vi "CRYO_MASTER_FULL_dev.vi"() -> ()   [LabVIEW 2017] (continued)
          }
          frame #2 {
            n644 = Search 1D Array(1D array=w1301, element="3He inlet pressure") -> (index of element=w1299:i32)  [unwired: 1 in]
            n645 = Index Array(array=w1300, index=w1299) -> (element=→"P_3HeIN" →"P (3He IN)":dbl)
          }
          frame #3 {
            n646 = Search 1D Array(1D array=w1306, element="Shield return press.") -> (index of element=w1304:i32)  [unwired: 1 in]
            n647 = Index Array(array=w1305, index=w1304) -> (element=→"P_SldRTN" →"P (shield return)":dbl)
          }
          frame #4 {
            n648 = Search 1D Array(1D array=w1311, element="3He pot pressure") -> (index of element=w1309:i32)  [unwired: 1 in]
            n649 = Index Array(array=w1310, index=w1309) -> (element=→"P_3Hepot" →"P (3He pot)":dbl)
          }
          frame #5 {
            n650 = Search 1D Array(1D array=w1316, element="1Kpot pressure") -> (index of element=w1313:i32)  [unwired: 1 in]
            n651 = Index Array(array=w1314, index=w1313) -> (element=→"P_1Kpot" →"P (1K pot)":dbl)
          }
          frame #6 {
            n652 = Search 1D Array(1D array=w1321, element="Dewar pressure") -> (index of element=w1318:i32)  [unwired: 1 in]
            n653 = Index Array(array=w1319, index=w1318) -> (element=→"P_Dewar" →"P (Dewar)":dbl)
          }
          frame #7 {
            n654 = Search 1D Array(1D array=w1326, element="HEX7 out pressure") -> (index of element=w1323:i32)  [unwired: 1 in]
            n655 = Index Array(array=w1324, index=w1323) -> (element=→"P_HEX7OUT" →"P (HEX7 out)":dbl)
          }
          frame #8 {
            n656 = Search 1D Array(1D array=w1331, element="Diff pressure HEX4") -> (index of element=w1328:i32)  [unwired: 1 in]
            n657 = Index Array(array=w1329, index=w1328) -> (element=→"DP_HEX4" →"DP HEX4":dbl)
          }
          frame #9 {
            n658 = Search 1D Array(1D array=w1336, element="Diff pressure HEX5") -> (index of element=w1333:i32)  [unwired: 1 in]
            n659 = Index Array(array=w1334, index=w1333) -> (element=→"DP_HEX5" →"DP HEX5":dbl)
          }
          frame #10 {
            n660 = Search 1D Array(1D array=w1341, element="3He pump exhaust flow") -> (index of element=w1338:i32)  [unwired: 1 in]
            n661 = Index Array(array=w1339, index=w1338) -> (element=→"F_1" →"F1 (3He pump exhaust) flow":dbl)
          }
          frame #11 {
            n662 = Search 1D Array(1D array=w1346, element="Shield flow") -> (index of element=w1343:i32)  [unwired: 1 in]
            n663 = Index Array(array=w1344, index=w1343) -> (element=→"F_2" →"F2 (shield flow)":dbl)
          }
          frame #12 {
            n664 = Search 1D Array(1D array=w1351, element="4He return flow from HEX7") -> (index of element=w1349:i32)  [unwired: 1 in]
            n665 = Index Array(array=w1348, index=w1349) -> (element=→"F_3" →"F3 (4He rtn flw via HEX7)":dbl)
          }
          frame #13 {
            n666 = Search 1D Array(1D array=w1356, element="3He incoming flow into HEX7") -> (index of element=w1354:i32)  [unwired: 1 in]
            n667 = Index Array(array=w1353, index=w1354) -> (element=→"F_4" →"F4 (3He in to HEX7)":dbl)
          }
          frame #14 {
            n668 = Search 1D Array(1D array=w1361, element="1Kpot pump exhaust flow") -> (index of element=w1359:i32)  [unwired: 1 in]
            n669 = Index Array(array=w1358, index=w1359) -> (element=→"F_5" →"F5 (1K pump ex.)":dbl)
          }
          frame #15 {
            n670 = Search 1D Array(1D array=w1366, element="4K reservoir level") -> (index of element=w1364:i32)  [unwired: 1 in]
            n671 = Index Array(array=w1363, index=w1364) -> (element=→"L3" →"He level (4K)":dbl)
          }
          frame #16 {
            n672 = Search 1D Array(1D array=w1371, element="1K pot level") -> (index of element=w1369:i32)  [unwired: 1 in]
            n673 = Index Array(array=w1368, index=w1369) -> (element=→"L(1K) (a1)" →"He level (1K)":dbl)
          }
          frame #17 {
            n674 = Search 1D Array(1D array=w1376, element="1K pot (b)") -> (index of element=w1374:i32)  [unwired: 1 in]
            n675 = Index Array(array=w1373, index=w1374) -> (element=→"1K pot(b1)" →"He level (1K) b":dbl)
          }
          frame #18 {
            n676 = case shown="False" TRUE {
              tunnel: w1381 -> [w1386 _]
              tunnel: "3He pot" -> [w1385 w1390]
              tunnel: w1379 -> [w1383 _]
              tunnel: [w1382 w1389] -> w1378
              frame False {
                n677 = Search 1D Array(1D array=w1386, element=w1385) -> (index of element=w1384:i32)  [unwired: 1 in]
                n678 = Index Array(array=w1383, index=w1384) -> (element=w1382:dbl)
              }
              frame True {
                n679 = local read "Labels (HP34401 LM)"() -> (w1391:string[])
                n680 = local read "LastData (HP34401 LM)"() -> (w1387:dbl[])
                n681 = Search 1D Array(1D array=w1391, element=w1390) -> (index of element=w1388:i32)  [unwired: 1 in]
                n682 = Index Array(array=w1387, index=w1388) -> (element=w1389:dbl)
              }
            }
            "3He pot level" <- w1378
            "He level (3He)" <- w1378
          }
        }
      }
    }
    n683 = case shown="True" w848 {
      tunnel: [w1952 w1964] -> w908
      tunnel: [w1942 w1963] -> w916
      tunnel: [w1951 w1962] -> w909
      tunnel: [w1950 timestamp[] [] ("TimeArray")] -> w878
      tunnel: [w1949 dbl[][] [] ("DataArray")] -> w876
      tunnel: w918 -> [w1948 w1959]
      tunnel: w917 -> [w1947 w1958]
      tunnel: w842 -> [w1943 _]
      tunnel: w845 -> [_ w1953]
      frame False {
        n684 = local read "Record interval"() -> (w1940:i64)
        n685 = call-dynamic "LSI336Data_measure.vi"("LSI336Data in"=w1948, "MeasurementIndex"=w1943, "error in (no error)"=w1947, "save every ... measurements"=w1940) -> ("Active?"=→"Active?\n(LSI336)":bool[], "TimeMeasuremeent"=→"Time of Last Measurement (LSI336)":timestamp, "LSI336Data out"=w1951:refnum<class "LSI336Data.lvclass">, "LastData"=→"Last Data \nLSI336":dbl[], "LastMeasurementConfig"=→"LastMeasurementConfig (336)":T17, "DataArray"=w1949:dbl[][], "Status"=w1942:u16, "TimeArray"=w1950:timestamp[], "error out"=w1952:errorcluster)  [unwired: 3 in]
      }
      frame True {
        n686 = local read "RUN Identifier"() -> (w1954:string)
        n687 = call-dynamic "LSI336Data_initialize.vi"("LSI336Data in"=w1959, "RunIdentifier"=w1954, "InstName"="InstName (LSI336)", "FileFormat"="FileFormat (336)", "LSI336Settings(X, Y)"="LSI336Settings(X,Y)", "error in (no error)"=w1958, "base path"=w1953) -> ("LSI336Data out"=w1962:refnum<class "LSI336Data.lvclass">, "Status"=w1963:T7, "AllLabels"=→"Labels LSI336":string[], "error out"=w1964:errorcluster)  [unwired: 5 in]
      }
    }
    "LSI336 Status" <- w916
    "error out (LSI336)" <- w908
    "TimeArray (LSI336)" <- w878
    "DataArray (336)" <- w876
    n688 = local read "Labels (HP34401 LM) 2"() -> (w841:string[])
    n689 = case shown="False" w848 {
      tunnel: [w2057 w2072] -> w921
      tunnel: [w2052 w2071] -> w938
      tunnel: [w2055 w2070] -> w922
      tunnel: w842 -> [w2056 _]
      tunnel: w937 -> [w2046 w2065]
      tunnel: w936 -> [w2047 w2064]
      tunnel: w845 -> [_ w2063]
      tunnel: [w2044 timestamp[] [] ("TimeArray")] -> w935
      tunnel: [w2043 dbl[][] [] ("DataArray")] -> w934
      frame False {
        w2050 = 24 ("index")
        n690 = local read "Record interval"() -> (w2041:i64)
        n691 = call-dynamic "LSI218Data_measure.vi"("LSI218Data in"=w2047, "MeasurementIndex"=w2056, "error in (no error)"=w2046, "save every ... measurements"=w2041) -> ("TimeMeasuremeent"=→"Time of Last Measurement (LSI218)":timestamp, "Active?"=w2051:bool[], "LSI218Data out"=w2055:refnum<class "LSI218Data.lvclass">, "LastMeasurementConfig"=→"LastMeasurementConfig (218)":T17, "LastData"=w2045:dbl[], "Status"=w2052:u16, "TimeArray"=w2044:timestamp[], "DataArray"=w2043:dbl[][], "error out"=w2057:errorcluster)  [unwired: 3 in]
        "LastData (LSI218)" <- w2045
        n692 = Split 1D Array(array=w2051, index=w2050) -> (first subarray=→"Active?\n (1)":bool[], second subarray=→"Active?\n(2)":bool[])
        n693 = Split 1D Array(array=w2045, index=w2050) -> (first subarray=→"Last Data \nLSI218 (1)":dbl[], second subarray=→"Last Data \nLSI218 (2)":dbl[])
      }
      frame True {
        n694 = local read "RUN Identifier"() -> (w2059:string)
        n695 = call-dynamic "LSI218Data_initialize.vi"("LSI218Settings(A-F)"="LSI218Settings(A-F)", "FileFormat"="FileFormat (218)", "base path"=w2063, "error in (no error)"=w2065, "InstName"="InstName (LSI218)", "RunIdentifier"=w2059, "LSI218Data in"=w2064) -> ("error out"=w2072:errorcluster, "Status"=w2071:T7, "AllLabels"=w2062:string[], "LSI218Data out"=w2070:refnum<class "LSI218Data.lvclass">)  [unwired: 1 in]
        n696 = Split 1D Array(array=w2062, index=24) -> (first subarray=→"Labels LSI218 (1)":string[], second subarray=→"Labels LSI218 (2)":string[])
      }
    }
    "LSI218 Status" <- w938
    "error out (LSI218)" <- w921
    n697 = case shown="False" w848 {
      tunnel: w847 -> [w1008 w1022]
      tunnel: [w1005 w1021] -> w846
      tunnel: w845 -> [_ w1019]
      tunnel: w844 -> [w1007 w1018]
      tunnel: [w1004 w1015] -> w843
      tunnel: w842 -> [w1006 _]
      tunnel: [w1002 dbl[][] [] ("LastDataArray")] -> w839
      tunnel: [w1001 timestamp[] [] ("LastTimeArray")] -> w837
      frame False {
        n698 = call-dynamic "LMData_measure.vi"("error in (no error)"=w1007, "MeasurementInterval(>0)"="LM measurement interval (>0)", "MeasurementIndex"=w1006, "LMData in"=w1008) -> ("error out"=w1004:errorcluster, "LastDataArray"=w1002:dbl[][], "LastMeasurement"=→"LastData (HP34401 LM)":dbl[], "LMData out"=w1005:refnum<class "LMData.lvclass">, "LastTimeArray"=w1001:timestamp[])  [unwired: 3 in]
      }
      frame True {
        n699 = local read "RUN Identifier"() -> (w1020:string)
        n700 = call-dynamic "LMData_initialize.vi"("LMData in"=w1022, "VISA resource name"="VISA (HP34401 LM)", "Labels"="Labels (HP34401 LM)", "FileFormat"="FileFormat (HP34401 LM)", "RunIdentifier"=w1020, "InstName"="InstName (HP34401 LM)", "base path"=w1019, "error in (no error)"=w1018, "LevelCalibration (R0, R1, L0, L1)"="LevelCalibration (R0, R1, L0, L1)", "Active?"="Active? (HP34401 LM)") -> ("LMData out"=w1021:refnum<class "LMData.lvclass">, "error out"=w1015:errorcluster)  [unwired: 4 in]
        "Labels (HP34401 LM) 2" <- "Labels (HP34401 LM)"
      }
    }
    "error out (HP34401 LM)" <- w843
    n701 = Array Size(array=w841) -> (size(s)=w840:i32)
    n702 = for {
      N: w840 -> [_]
      tunnel: w839 -> [w962]
      shift-right: [w949] -> w833
      shift-left: w838 -> [w948]
      shift-right: [w952] -> w835
      shift-left: w838 -> [w953]
      shift-right: [w956] -> w836
      shift-left: w838 -> [w957]
      shift-right: [w951] -> w834
      shift-left: w838 -> [w950]
      tunnel: w837 -> [w960]
      i -> [w961]
      n703 = local read "Plot selecter (HP34401A)\n    1      2     3     4"() -> (w967:bool[][])
      n704 = Index Array(array=w962, index (col)=w961) -> (element=w959:dbl[])  [unwired: 1 in]
      n705 = Bundle("LastTimeArray"=w960, "LastDataArray"=w959) -> (w958:T29)  [unwired: 1 in]
      n706 = Index Array(array=w967, index (row) #1=w961, index (col) #1=0 ("disabled index (col)"), index (row) #2=w961, index (col) #2=1 ("index (col)"), index (row) #3=w961, index (col) #3=2 ("index (col)"), index (row) #4=w961, index (col) #4=3 ("disabled index (col)")) -> (element #1=w955:bool, element #2=w954:bool)  [unwired: 2 out]
      n707 = stacked-sequence {
        tunnel: w958 -> [w969 w976 w986 w994]
        tunnel: w957 -> [w971 _ _ _]
        tunnel: [w970 _ _ _] -> w956
        tunnel: w955 -> [w968 _ _ _]
        tunnel: w954 -> [_ w979 w987 w995]
        tunnel: w953 -> [_ w978 _ _]
        tunnel: [_ w977 _ _] -> w952
        tunnel: [_ _ w985 _] -> w951
        tunnel: w950 -> [_ _ w984 _]
        tunnel: [_ _ _ w993] -> w949
        tunnel: w948 -> [_ _ _ w992]
        frame #0 {
          n708 = case shown="False" w968 {
            tunnel: w971 -> [w972 w975]
            tunnel: [w972 w974] -> w970
            tunnel: w969 -> [_ w973]
            frame False {
            }
            frame True {
              n709 = Build Array (concatenate)(w975, w973) -> (w974:T30)
            }
          }
        }
        frame #1 {
          n710 = case shown="False" w979 {
            tunnel: [w980 w983] -> w977
            tunnel: w978 -> [w980 w982]
            tunnel: w976 -> [_ w981]
            frame False {
            }
            frame True {
              n711 = Build Array (concatenate)(w982, w981) -> (w983:T30)
            }
          }
        }
        frame #2 {
          n712 = case shown="False" w987 {
            tunnel: [w988 w991] -> w985
            tunnel: w986 -> [_ w990]
            tunnel: w984 -> [w988 w989]
            frame False {
            }
            frame True {
              n713 = Build Array (concatenate)(w989, w990) -> (w991:T30)
            }
          }
        }
        frame #3 {
          n714 = case shown="True" w995 {
            tunnel: [w996 w999] -> w993
            tunnel: w994 -> [_ w998]
            tunnel: w992 -> [w996 w997]
            frame False {
            }
            frame True {
              n715 = Build Array (concatenate)(w997, w998) -> (w999:T30)
            }
          }
        }
      }
    }
    n716 = local read "Last Data \n(USB6210)"() -> (w862:dbl[])
    n717 = local read "Last Data \n(USB6218)"() -> (w863:dbl[])
    n718 = local read "All Labels (USB6210)"() -> (w865:string[])
    n719 = local read "All Labels (USB6218)"() -> (w864:string[])
    n720 = flat-sequence {
      tunnel: w892 -> [w1450]
      tunnel: [w1445] -> w891
      tunnel: [w1443] -> w890
      tunnel: [w1442] -> w889
      tunnel: [w1441] -> w888
      tunnel: w893 -> [w1437]
      frame #0 {
        w1444 = T25 [] ("appended array")
        n721 = Unbundle By Name(w1437) -> ("TimeArray"=w1433:timestamp[], "DataArrayConv"=w1448:dbl[][], "LDArray"=w1447:dbl[])
        "TimeArray (USB6218)" <- w1433
        n722 = Unbundle By Name(w1450) -> ("ReadLeakDet?"=w1449:bool, "LabelLD"=w1452:string, "Labels"=w1446:string[])  [unwired: 1 out]
        n723 = case shown="True" w1449 {
          tunnel: w1452 -> [_ w1460]
          tunnel: w1448 -> [w1454 w1459]
          tunnel: w1447 -> [_ w1458]
          tunnel: [w1454 w1457] -> w1435
          tunnel: w1446 -> [w1453 w1456]
          tunnel: [w1453 w1455] -> w1438
          frame False {
          }
          frame True {
            n724 = Build Array (concatenate)(w1459, w1458) -> (w1457:dbl[][])
            n725 = Build Array (concatenate)(w1456, w1460) -> (w1455:string[])
          }
        }
        "All Labels (USB6218)" <- w1438
        "DataArrayConv (USB6218)" <- w1435
        n726 = Array Size(array=w1433) -> (size(s)=→"TimeArray size (6218)":i32)
        n727 = local read "Plot selecter (USB6218)\n    1      2     3     4"() -> (w1440:bool[][])
        n728 = control-ref of="Plot selecter (USB6218)\n    1      2     3     4"() -> (w1436:refnum<vi>)
        n729 = Array Size(array=w1438) -> (size(s)=w1439:i32)
        n730 = Array Size(array=w1438) -> (size(s)=w1451:i32)
        n731 = Array Size(array=w1435) -> (size(s)=→"DataArraySize (6218)":i32[])
        n732 = property on="Property Node" class="Arr (strict)"(reference=w1436, "Number of Rows"=w1439) -> ()  [unwired: 1 in, 2 out]
        n733 = for {
          N: w1451 -> [_]
          tunnel: w1435 -> [w1481]
          tunnel: w1433 -> [w1482]
          shift-right: [w1476] -> w1443
          shift-left: w1444 -> [w1479]
          shift-right: [w1474] -> w1441
          shift-left: w1444 -> [w1477]
          shift-right: [w1475] -> w1445
          shift-left: w1444 -> [w1473]
          shift-right: [w1472] -> w1442
          shift-left: w1444 -> [w1471]
          tunnel: w1440 -> [w1470]
          i -> [w1465]
          n734 = Index Array(array=w1481, index (col)=w1465) -> (element=w1480:dbl[])  [unwired: 1 in]
          n735 = Index Array(array=w1470, index (row) #1=w1465, index (col) #1=0 ("index (row)"), index (row) #2=w1465, index (col) #2=1 ("index (row)"), index (row) #3=w1465, index (col) #3=2 ("index (row)"), index (row) #4=w1465, index (col) #4=3 ("index (row)")) -> (element #1=w1464:bool, element #2=w1463:bool, element #3=w1462:bool, element #4=w1461:bool)
          n736 = Bundle("TimeArray"=w1482, "DataArrayConv"=w1480) -> (w1478:T31)  [unwired: 1 in]
          n737 = stacked-sequence {
            tunnel: w1464 -> [w1486 _ _ _]
            tunnel: w1479 -> [_ w1494 _ _]
            tunnel: w1462 -> [_ _ w1502 _]
            tunnel: w1478 -> [w1483 w1492 w1501 w1507]
            tunnel: w1461 -> [_ _ _ w1510]
            tunnel: w1477 -> [_ _ _ w1509]
            tunnel: [_ _ _ w1508] -> w1474
            tunnel: [_ w1493 _ _] -> w1476
            tunnel: [w1485 _ _ _] -> w1475
            tunnel: w1473 -> [w1484 _ _ _]
            tunnel: [_ _ w1500 _] -> w1472
            tunnel: w1471 -> [_ _ w1499 _]
            tunnel: w1463 -> [_ w1491 _ _]
            frame #0 {
              n738 = case shown="True" w1486 {
                tunnel: [w1487 w1490] -> w1485
                tunnel: w1483 -> [_ w1489]
                tunnel: w1484 -> [w1487 w1488]
                frame False {
                }
                frame True {
                  n739 = Build Array (concatenate)(w1488, w1489) -> (w1490:T25)
                }
              }
            }
            frame #1 {
              n740 = case shown="True" w1491 {
                tunnel: w1494 -> [w1495 w1498]
                tunnel: [w1495 w1497] -> w1493
                tunnel: w1492 -> [_ w1496]
                frame False {
                }
                frame True {
                  n741 = Build Array (concatenate)(w1498, w1496) -> (w1497:T25)
                }
              }
            }
            frame #2 {
              n742 = case shown="True" w1502 {
                tunnel: [w1503 w1506] -> w1500
                tunnel: w1501 -> [_ w1505]
                tunnel: w1499 -> [w1503 w1504]
                frame False {
                }
                frame True {
                  n743 = Build Array (concatenate)(w1504, w1505) -> (w1506:T25)
                }
              }
            }
            frame #3 {
              n744 = case shown="True" w1510 {
                tunnel: [w1511 w1514] -> w1508
                tunnel: w1507 -> [_ w1513]
                tunnel: w1509 -> [w1511 w1512]
                frame False {
                }
                frame True {
                  n745 = Build Array (concatenate)(w1512, w1513) -> (w1514:T25)
                }
              }
            }
          }
        }
      }
    }
    n746 = case shown="True" "Digital Out ON?" {
      tunnel: w848 -> [_ w1653]
      tunnel: w898 -> [w1647 w1652]
      tunnel: [w1647 w1651] -> w897
      tunnel: w896 -> [_ w1650]
      tunnel: w845 -> [_ w1649]
      tunnel: w879 -> [_ w1648]
      frame False {
      }
      frame True {
        n747 = case shown="True" w1653 {
          tunnel: w1652 -> [w1671 w1854]
          tunnel: [w1671 w1867] -> w1651
          tunnel: w1650 -> [w1672 _]
          tunnel: w1649 -> [_ w1846]
          tunnel: w1648 -> [_ _]
          frame False {
            n748 = flat-sequence {
              frame #0 {
              }
            }
            n749 = case shown="\"USB6218AI\"" "AutoFill Source (P)" {
              tunnel: [w1675 w1676] -> w1657
              frame "USB6210", Default {
                n750 = local read "All Labels (USB6210)"() -> (w1675:string[])
              }
              frame "USB6218AI" {
                n751 = local read "All Labels (USB6218)"() -> (w1676:string[])
              }
            }
            n752 = case shown="\"USB6210\", Default" "AutoFill Source (L)" {
              tunnel: [w1673 w1674] -> w1654
              frame "USB6210", Default {
                n753 = local read "All Labels (USB6210)"() -> (w1673:string[])
              }
              frame "USB6218AI" {
                n754 = local read "All Labels (USB6218)"() -> (w1674:string[])
              }
            }
            n755 = Multiply(x="N for sampling", y=i64 2) -> (x*y=w1666:i64)
            n756 = local read "Cycle #"() -> (w1670:u32)
            n757 = Search 1D Array(1D array=w1657, element="Auto Fll Dewar P. label") -> (index of element=→"Target Index (P)":i32)  [unwired: 1 in]
            n758 = Search 1D Array(1D array=w1654, element="Auto Fll He L. label") -> (index of element=→"Target Index (L)":i32)  [unwired: 1 in]
            n759 = Add(x=w1666, y="Mov. Avg Interval") -> (x+y=w1668:i64)
            n760 = Greater?(x=w1670, y=w1668) -> (0:w1664:bool)
            n761 = And(x=w1664, y="Auto Fill ON?") -> (x .and. y?=w1662:bool)
            n762 = case shown="True" w1662 {
              tunnel: w1672 -> [_ w1710]
              tunnel: "Mov. Avg Interval" -> [_ w1696]
              tunnel: w1666 -> [_ w1683]
              tunnel: "N for sampling" -> [_ w1694]
              frame False {
              }
              frame True {
                n763 = local read "AutoFill Source (L)"() -> (w1677:T8)
                n764 = local read "AutoFill Source (P)"() -> (w1678:T8)
                n765 = case shown="\"USB6218AI\"" w1678 {
                  tunnel: [w1714 w1715] -> w1679
                  frame "USB6210", Default {
                    n766 = local read "DataArrayConv (USB6210)"() -> (w1714:dbl[][])
                  }
                  frame "USB6218AI" {
                    n767 = local read "DataArrayConv (USB6218)"() -> (w1715:dbl[][])
                  }
                }
                n768 = case shown="\"USB6210\", Default" w1677 {
                  tunnel: [w1712 w1713] -> w1681
                  frame "USB6210", Default {
                    n769 = local read "DataArrayConv (USB6210)"() -> (w1712:dbl[][])
                  }
                  frame "USB6218AI" {
                    n770 = local read "DataArrayConv (USB6218)"() -> (w1713:dbl[][])
                  }
                }
                n771 = local read "Pstd"() -> (→"Pstd history":dbl)
                n772 = local read "Lstd"() -> (→"Lstd history":dbl)
                n773 = local read "Target Index (L)"() -> (w1682:i32)
                n774 = local read "Pav (Pa)"() -> (→"Pav history":dbl)
                n775 = local read "Lav (%)"() -> (→"Lav history":dbl)
                n776 = Index Array(array=w1681, index (col)=w1682) -> (element=w1680:dbl[])  [unwired: 1 in]
                n777 = local read "Target Index (P)"() -> (w1711:i32)
                n778 = Unbundle By Name(w1710) -> ("TimeArray"=w1709:timestamp[])
                n779 = Index Array(array=w1679, index (col)=w1711) -> (element=w1698:dbl[])  [unwired: 1 in]
                n780 = Delete From Array(array=w1698, length=w1683) -> (deleted portion=w1706:dbl[])  [unwired: 1 in, 1 out]
                n781 = Delete From Array(array=w1680, length=w1683) -> (deleted portion=w1693:dbl[])  [unwired: 1 in, 1 out]
                n782 = call "MovingAverage.vi"("Moving Average interval"=w1696, "Input Array"=w1680) -> ("M.A. Array"=w1695:dbl[])  [unwired: 9 in]
                n783 = call "MovingAverage.vi"("Moving Average interval"=w1696, "Input Array"=w1698) -> ("M.A. Array"=w1697:dbl[])  [unwired: 9 in]
                n784 = Delete From Array(array=w1697, length=w1683) -> (deleted portion=w1707:dbl[])  [unwired: 1 in, 1 out]
                n785 = Delete From Array(array=w1697, length=w1683) -> (deleted portion=w1703:dbl[])  [unwired: 1 in, 1 out]
                "Last N M.A. Pressures" <- w1703
                n786 = Delete From Array(array=w1695, length=w1683) -> (deleted portion=w1688:dbl[])  [unwired: 1 in, 1 out]
                "Last N M.A. Levels" <- w1688
                n787 = Delete From Array(array=w1709, length=w1683) -> (deleted portion=w1690:timestamp[])  [unwired: 1 in, 1 out]
                n788 = Bundle("TimeArray"=w1690, "DataArrayConv (USB6218)"=w1706) -> (w1705:T32)  [unwired: 1 in]
                n789 = Bundle("TimeArray"=w1690, "M.A. Array"=w1707) -> (w1708:T33)  [unwired: 1 in]
                n790 = Bundle("TimeArray"=w1690, "DataArrayConv (USB6218)"=w1693) -> (w1692:T32)  [unwired: 1 in]
                n791 = Bundle("TimeArray"=w1690, "M.A. Array"=w1688) -> (w1689:T33)  [unwired: 1 in]
                n792 = Array Size(array=w1703) -> (size(s)=w1702:i32)
                n793 = Greater Or Equal?(x=w1702, y=w1694) -> (x >= y?=w1701:bool)
                n794 = Build Array(w1705, w1708) -> (→"Dewar Pressure":T34)
                n795 = Build Array(w1692, w1689) -> (→"He Level":T34)
                n796 = case shown="True" w1701 {
                  tunnel: [w1819 w1824] -> w1687
                  tunnel: w1703 -> [_ w1825]
                  tunnel: w1688 -> [_ w1822]
                  tunnel: [w1819 w1820] -> w1686
                  frame False {
                    w1819 = nan ("mean")
                  }
                  frame True {
                    n797 = call <vilib>:"Std Deviation and Variance.vi"("X"=w1825) -> ("mean"=w1824:dbl, "standard deviation"=w1823:dbl)  [unwired: 1 in, 1 out]
                    n798 = call <vilib>:"Std Deviation and Variance.vi"("X"=w1822) -> ("mean"=w1820:dbl, "standard deviation"=w1821:dbl)  [unwired: 1 in, 1 out]
                    n799 = local write "Pstd"(w1823) -> ()
                    n800 = local write "Lstd"(w1821) -> ()
                    n801 = local write "Pav (Pa)"(w1824) -> ()
                    n802 = local write "Lav (%)"(w1820) -> ()
                  }
                }
                n803 = flat-sequence {
                  tunnel: w1687 -> [w1716]
                  tunnel: w1686 -> [w1717]
                  frame #0 {
                    n804 = flat-sequence {
                      tunnel: w1717 -> [w1719]
                      tunnel: w1716 -> [w1718]
                      tunnel: w1716 -> [w1787]
                      frame #0 {
                        n805 = stacked-sequence {
                          tunnel: w1719 -> [w1726 w1730 _ _ _ _]
                          tunnel: w1718 -> [_ _ w1744 w1753 w1762 w1771]
                          frame #0 {
                            n806 = local read "L_low (%)"() -> (w1725:dbl)
                            n807 = local read "Fill state"() -> (w1723:bool)
                            n808 = Less?(x=w1726, y=w1725) -> (x < y?=w1722:bool)
                            n809 = Equal?(x=w1723, y=FALSE) -> (x = y?=w1721:bool)
                            n810 = And(x=w1722, y=w1721) -> (x .and. y?=w1720:bool)
                            n811 = case shown="False" w1720 {
                              frame False {
                              }
                              frame True {
                                w1728 = TRUE ("Value (Signaling)")
                                n812 = property on="Fill state" class="Bool (strict)"("Val(Sgnl)"=w1728) -> ()  [unwired: 2 in, 2 out]
                                n813 = Not(x=w1728) -> (.not. x?=w1727:bool)
                                n814 = property on="Fill (false)" class="Bool (strict)"("Val(Sgnl)"=w1727) -> ()  [unwired: 2 in, 2 out]
                              }
                            }
                          }
                          frame #1 {
                            n815 = local read "L_high (%)"() -> (w1731:dbl)
                            n816 = local read "Fill state"() -> (w1734:bool)
                            n817 = Greater?(x=w1730, y=w1731) -> (0:w1729:bool)
                            n818 = Equal?(x=w1734, y=TRUE) -> (x = y?=w1733:bool)
                            n819 = And(x=w1729, y=w1733) -> (x .and. y?=w1732:bool)
                            n820 = case shown="True" w1732 {
                              frame False {
                              }
                              frame True {
                                w1736 = FALSE ("Value (Signaling)")
                                n821 = property on="Fill state" class="Bool (strict)"("Val(Sgnl)"=w1736) -> ()  [unwired: 2 in, 2 out]
                                n822 = Not(x=w1736) -> (.not. x?=w1737:bool)
                                n823 = property on="Fill (false)" class="Bool (strict)"("Val(Sgnl)"=w1737) -> ()  [unwired: 2 in, 2 out]
                              }
                            }
                          }
                          frame #2 {
                            n824 = local read "P_1_low (Pa)"() -> (w1743:dbl)
                            n825 = property on="state 1" class="Bool (strict)"() -> ("Value"=w1741:bool)  [unwired: 2 in, 2 out]
                            n826 = Less?(x=w1744, y=w1743) -> (x < y?=w1740:bool)
                            n827 = Equal?(x=w1741, y=FALSE) -> (x = y?=w1739:bool)
                            n828 = And(x=w1739, y=w1740) -> (x .and. y?=w1738:bool)
                            n829 = case shown="True" w1738 {
                              frame False {
                              }
                              frame True {
                                w1746 = TRUE ("Value (Signaling)")
                                n830 = property on="state 1" class="Bool (strict)"("Val(Sgnl)"=w1746) -> ()  [unwired: 2 in, 2 out]
                                n831 = Not(x=w1746) -> (.not. x?=w1745:bool)
                                n832 = property on="state 1 (false)" class="Bool (strict)"("Val(Sgnl)"=w1745) -> ()  [unwired: 2 in, 2 out]
                              }
                            }
                          }
                          frame #3 {
                            n833 = local read "P_1_high (Pa)"() -> (w1752:dbl)
                            n834 = property on="state 1" class="Bool (strict)"() -> ("Value"=w1750:bool)  [unwired: 2 in, 2 out]
                            n835 = Greater?(x=w1753, y=w1752) -> (0:w1749:bool)
                            n836 = Equal?(x=w1750, y=TRUE) -> (x = y?=w1748:bool)
                            n837 = And(x=w1748, y=w1749) -> (x .and. y?=w1747:bool)
                            n838 = case shown="True" w1747 {
                              frame False {
                              }
                              frame True {
                                w1755 = FALSE ("Value (Signaling)")
                                n839 = property on="state 1" class="Bool (strict)"("Val(Sgnl)"=w1755) -> ()  [unwired: 2 in, 2 out]
                                n840 = Not(x=w1755) -> (.not. x?=w1754:bool)
                                n841 = property on="state 1 (false)" class="Bool (strict)"("Val(Sgnl)"=w1754) -> ()  [unwired: 2 in, 2 out]
                              }
                            }
                          }
                          frame #4 {
                            n842 = local read "P_2_low (Pa)"() -> (w1761:dbl)
                            n843 = property on="state 2" class="Bool (strict)"() -> ("Value"=w1756:bool)  [unwired: 2 in, 2 out]
                            n844 = Less?(x=w1762, y=w1761) -> (x < y?=w1759:bool)
                            n845 = Equal?(x=w1756, y=FALSE) -> (x = y?=w1758:bool)
                            n846 = And(x=w1758, y=w1759) -> (x .and. y?=w1757:bool)
                            n847 = case shown="True" w1757 {
                              frame False {
                              }
                              frame True {
                                w1763 = TRUE ("Value (Signaling)")
                                n848 = property on="state 2" class="Bool (strict)"("Val(Sgnl)"=w1763) -> ()  [unwired: 2 in, 2 out]
                                n849 = Not(x=w1763) -> (.not. x?=w1764:bool)
                                n850 = property on="state 2 (false)" class="Bool (strict)"("Val(Sgnl)"=w1764) -> ()  [unwired: 2 in, 2 out]
                              }
                            }
                          }
                          frame #5 {
                            n851 = local read "P_2_high (Pa)"() -> (w1770:dbl)
                            n852 = property on="state 2" class="Bool (strict)"() -> ("Value"=w1765:bool)  [unwired: 2 in, 2 out]
                            n853 = Greater?(x=w1771, y=w1770) -> (0:w1768:bool)
                            n854 = Equal?(x=w1765, y=TRUE) -> (x = y?=w1767:bool)
                            n855 = And(x=w1767, y=w1768) -> (x .and. y?=w1766:bool)
                            n856 = case shown="True" w1766 {
                              frame False {
                              }
                              frame True {
                                w1772 = FALSE ("Value (Signaling)")
                                n857 = property on="state 2" class="Bool (strict)"("Val(Sgnl)"=w1772) -> ()  [unwired: 2 in, 2 out]
                                n858 = Not(x=w1772) -> (.not. x?=w1773:bool)
                                n859 = property on="state 2 (false)" class="Bool (strict)"("Val(Sgnl)"=w1773) -> ()  [unwired: 2 in, 2 out]
                              }
                            }
                          }
                        }
                      }
                      frame #1 {
                        n860 = property on="Fill state" class="Bool (strict)"() -> ("Value"=w1774:bool)  [unwired: 2 in, 2 out]
                        n861 = case shown="True" w1774 {
                          frame False {
                            n862 = property on="V1 (N.O.)" class="Bool (strict)"("Val(Sgnl)"=TRUE ("V1 (N.O.)")) -> ()  [unwired: 2 in, 2 out]
                            n863 = property on="V2 (N.C.)" class="Bool (strict)"("Val(Sgnl)"=FALSE ("Value (Signaling)")) -> ()  [unwired: 2 in, 2 out]
                          }
                          frame True {
                            n864 = property on="state 1" class="Bool (strict)"() -> ("Value"=w1778:bool)  [unwired: 2 in, 2 out]
                            n865 = property on="state 2" class="Bool (strict)"() -> ("Value"=w1777:bool)  [unwired: 2 in, 2 out]
                            n866 = case shown="True" w1778 {
                              frame False {
                                n867 = property on="V1 (N.O.)" class="Bool (strict)"("Val(Sgnl)"=TRUE ("Value (Signaling)")) -> ()  [unwired: 2 in, 2 out]
                                n868 = local write "Status V1 CTRL"(enum16{"Pressurize", "Release"}."Release" ("Status V1 CTRL")) -> ()
                              }
                              frame True {
                                n869 = property on="V1 (N.O.)" class="Bool (strict)"("Val(Sgnl)"=FALSE ("V1 (N.O.)")) -> ()  [unwired: 2 in, 2 out]
                                n870 = local write "Status V1 CTRL"(enum16{"Pressurize", "Release"}."Pressurize" ("Status V1 CTRL")) -> ()
                              }
                            }
                            n871 = case shown="True" w1777 {
                              frame False {
                                n872 = property on="V2 (N.C.)" class="Bool (strict)"("Val(Sgnl)"=FALSE ("Value (Signaling)")) -> ()  [unwired: 2 in, 2 out]
                                n873 = local write "Status V2 CTRL"(enum16{"Pressurize", "Release"}."Release" ("Status V2 CTRL")) -> ()
                              }
                              frame True {
                                n874 = property on="V2 (N.C.)" class="Bool (strict)"("Val(Sgnl)"=TRUE ("Value (Signaling)")) -> ()  [unwired: 2 in, 2 out]
                                n875 = local write "Status V2 CTRL"(enum16{"Pressurize", "Release"}."Pressurize" ("Status V2 CTRL")) -> ()
                              }
                            }
                          }
                        }
                      }
                      frame #2 {
                        n876 = Greater?(x=w1787, y="P_safelimit_high (Pa)") -> (0:w1789:bool)
                        n877 = Less?(x=w1787, y="P_safelimit_low (Pa)") -> (x < y?=w1791:bool)
                        n878 = Or(x=w1789, y=w1791) -> (x .or. y?=w1792:bool)
                        n879 = case shown="False" w1792 {
                          frame False {
                          }
                          frame True {
                            w1793 = FALSE ("Value (Signaling)")
                            w1795 = FALSE ("Value (Signaling)")
                            n880 = property on="V2 (N.C.)" class="Bool (strict)"("Val(Sgnl)"=FALSE ("V1 (N.O.)")) -> ()  [unwired: 2 in, 2 out]
                            n881 = property on="state 1" class="Bool (strict)"("Val(Sgnl)"=w1793) -> ()  [unwired: 2 in, 2 out]
                            n882 = property on="V1 (N.O.)" class="Bool (strict)"("Val(Sgnl)"=TRUE ("V1 (N.O.)")) -> ()  [unwired: 2 in, 2 out]
                            n883 = property on="state 2" class="Bool (strict)"("Val(Sgnl)"=w1795) -> ()  [unwired: 2 in, 2 out]
                            n884 = Not(x=w1793) -> (.not. x?=w1794:bool)
                            n885 = Not(x=w1795) -> (.not. x?=w1796:bool)
                            n886 = property on="state 1 (false)" class="Bool (strict)"("Val(Sgnl)"=w1794) -> ()  [unwired: 2 in, 2 out]
                            n887 = property on="state 2 (false)" class="Bool (strict)"("Val(Sgnl)"=w1796) -> ()  [unwired: 2 in, 2 out]
                          }
                        }
                      }
                    }
                  }
                  frame #1 {
                    n888 = property on="V2 (N.C.)" class="Bool (strict)"() -> ("Value"=w1806:bool)  [unwired: 2 in, 2 out]
                    n889 = property on="V1 (N.O.)" class="Bool (strict)"() -> ("Value"=w1817:bool)  [unwired: 2 in, 2 out]
                    n890 = local read "P_1_high (Pa)"() -> (w1811:dbl)
                    n891 = local read "P_2_high (Pa)"() -> (w1809:dbl)
                    n892 = local read "P_1_low (Pa)"() -> (w1812:dbl)
                    n893 = local read "P_2_low (Pa)"() -> (w1810:dbl)
                    n894 = local read "L_high (%)"() -> (w1807:dbl)
                    n895 = local read "L_low (%)"() -> (w1808:dbl)
                    n896 = local read "Pav (Pa)"() -> (w1800:dbl)
                    n897 = local read "Lav (%)"() -> (w1799:dbl)
                    n898 = Boolean To (0,1)(Boolean=w1806) -> (0, 1=w1805:i16)
                    n899 = Boolean To (0,1)(Boolean=w1817) -> (0, 1=w1818:i16)
                    n900 = local read "File Refn DewarCTRL"() -> (w1813:refnum<file>)
                    n901 = local read "Cycle #"() -> (w1816:u32)
                    n902 = Build Array(w1800, w1799, w1812, w1811, w1810, w1809, w1808, w1807, w1818, w1805) -> (w1804:dbl[])
                    n903 = Get Date/Time In Seconds() -> (seconds since 1Jan1904=w1814:timestamp)
                    n904 = call "FileWrite.vi"("DataArray"=w1804, "Time Stamp"=w1814, "Error In"=errorcluster {"status"=FALSE, "code"=0, "source"=""}, "FileFormat"=string[] ["%4.5e", "%4.2f", "%4.4e", "%4.4e", "%4.4e", "%4.4e", "%4.4e", "%d", "%d"] ("Array"), "Index"=w1816, "refnum in"=w1813) -> ("Error Out"=→"Error Out (Dewar CTRL":errorcluster, "Byte Stream File Refnum"=w1803:refnum<file>)  [unwired: 4 in]
                    n905 = local write "File Refn DewarCTRL"(w1803) -> ()
                  }
                }
              }
            }
          }
          frame True {
            w1864 = "_"
            w1827 = FALSE ("auto cleanup")
            w1829 = 1 items=["one channel for each line", "one channel for all lines"] ("line grouping")
            n906 = flat-sequence {
              frame #0 {
                w1881 = FALSE ("V1 (N.O.)")
                n907 = local write "V1 (N.O.)"(TRUE ("V1 (N.O.)")) -> ()
                n908 = local write "V2 (N.C.)"(FALSE ("V1 (N.O.)")) -> ()
                n909 = local write "state 2"(w1881) -> ()
                n910 = local write "state 1"(w1881) -> ()
                n911 = local write "Fill state"(w1881) -> ()
                n912 = Not(x=w1881) -> (.not. x?=w1883:bool)
                n913 = Not(x=w1881) -> (.not. x?=w1882:bool)
                n914 = local write "state 1 (false)"(w1882) -> ()
                n915 = local write "state 2 (false)"(w1882) -> ()
                n916 = local write "Fill (false)"(w1883) -> ()
              }
            }
            n917 = Get Date/Time In Seconds() -> (seconds since 1Jan1904=w1878:timestamp)
            n918 = call "LV_UNIXTIME.vi"("current time"=w1878) -> ("date/time string"=w1859:string)  [unwired: 9 in, 1 out]
            n919 = local read "RUN Identifier"() -> (w1826:string)
            n920 = Concatenate Strings(w1859, "_DO" ("new task name")) -> (w1875:string)
            n921 = Concatenate Strings(w1826, w1864, w1859, w1864) -> (w1845:string)
            n922 = Concatenate Strings(w1845, "DEWAR.csv" ("string")) -> (w1844:string)
            n923 = Concatenate Strings(w1845, "USB_DOUT.csv" ("string")) -> (w1848:string)
            n924 = Build Path(base path=w1846, name or relative path=w1844) -> (appended path=w1843:path)
            n925 = Build Path(base path=w1846, name or relative path=w1848) -> (appended path=w1863:path)
            n926 = Open/Create/Replace File(file path (use dialog)=w1863, error in=w1854, operation (0:open)=T24."open or create") -> (refnum out=w1861:refnum<file>, error out=w1853:errorcluster)  [unwired: 3 in, 1 out]
            n927 = call "FileIntialize.vi"("Error In"=w1853, "Labels"="DOUT Labels", "refnum in"=w1861) -> ("Error Out"=w1840:errorcluster, "File Refnum"=→"File Refn USB DO":refnum<file>)  [unwired: 7 in]
            n928 = Open/Create/Replace File(file path (use dialog)=w1843, error in=w1840, operation (0:open)=T24."open or create") -> (refnum out=w1851:refnum<file>, error out=w1852:errorcluster)  [unwired: 3 in, 1 out]
            n929 = call "FileIntialize.vi"("Error In"=w1852, "Labels"=string[] ["P_av", "L_av", "P_1_low", "P_1_high", "P_2_low", "P_2_high", "L_low", "L_high", "V1(NO)", "V2(NC)"], "refnum in"=w1851) -> ("Error Out"=w1839:errorcluster, "File Refnum"=→"File Refn DewarCTRL":refnum<file>)  [unwired: 7 in]
            n930 = Index Array(array="DOUT Physical CH", index #1=0 ("index"), index #2=1 ("index"), index #3=2 ("index"), index #4=3 ("index")) -> (element #1=w1857:tag, element #2=w1835:tag, element #3=w1834:tag, element #4=w1828:tag)
            n931 = call <vilib>:"DAQmx Create Task.vi"("new task name"=w1875, "auto cleanup"=FALSE, "error in"=w1839) -> ("task out"=w1876:refnum<k21>, "error out"=w1877:errorcluster)  [unwired: 11 in]
            n932 = call-poly <vilib>:"DAQmx Create Virtual Channel.vi"("task in"=w1876, "lines"=w1857, "line grouping"=w1829, "error in"=w1877) -> ("task out"=w1879:refnum<k21>, "error out"=w1880:errorcluster)  [unwired: 10 in]
            n933 = call-poly <vilib>:"DAQmx Create Virtual Channel.vi"("task in"=w1879, "lines"=w1835, "line grouping"=w1829, "error in"=w1880) -> ("task out"=w1866:refnum<k21>, "error out"=w1865:errorcluster)  [unwired: 10 in]
            n934 = call-poly <vilib>:"DAQmx Create Virtual Channel.vi"("task in"=w1866, "lines"=w1834, "line grouping"=w1829, "error in"=w1865) -> ("task out"=w1833:refnum<k21>, "error out"=w1832:errorcluster)  [unwired: 10 in]
            n935 = call-poly <vilib>:"DAQmx Create Virtual Channel.vi"("task in"=w1833, "lines"=w1828, "line grouping"=w1829, "error in"=w1832) -> ("task out"=w1830:refnum<k21>, "error out"=w1831:errorcluster)  [unwired: 10 in]
            n936 = call <vilib>:"DAQmx Start Task.vi"("task/channels in"=w1830, "error in"=w1831) -> ("task out"=w1870:refnum<k21>, "error out"=w1868:errorcluster)  [unwired: 12 in]
            n937 = Build Array(w1827, w1827, w1827, w1827) -> (w1871:bool[])
            n938 = call <vilib>:"DAQmx Write (Digital 1D Bool NChan 1Samp 1Line).vi"("task/channels in"=w1870, "data"=w1871, "timeout"=10.0, "error in"=w1868) -> ("task out"=→"DOUT task out":refnum<k21>, "error out"=w1867:errorcluster)  [unwired: 9 in, 1 out]
          }
        }
      }
    }
    "error out (USB6210/6218 DOUT)" <- w897
    n939 = Build Array (concatenate)(w862, w863) -> (w860:dbl[])
    n940 = Build Array (concatenate)(w865, w864) -> (w861:string[])
    n941 = flat-sequence {
      tunnel: w944 -> [w1531]
      tunnel: [w1526] -> w932
      tunnel: [w1524] -> w930
      tunnel: [w1523] -> w927
      tunnel: [w1522] -> w925
      tunnel: w896 -> [w1517]
      frame #0 {
        w1525 = T25 [] ("appended array")
        n942 = Unbundle By Name(w1517) -> ("TimeArray"=w1534:timestamp[], "DataArrayConv"=w1529:dbl[][], "LDArray"=w1528:dbl[])
        n943 = Unbundle By Name(w1531) -> ("ReadLeakDet?"=w1530:bool, "LabelLD"=w1533:string, "Labels"=w1527:string[])  [unwired: 1 out]
        n944 = case shown="True" w1530 {
          tunnel: w1533 -> [_ w1542]
          tunnel: w1529 -> [w1536 w1541]
          tunnel: w1528 -> [_ w1540]
          tunnel: [w1536 w1539] -> w1516
          tunnel: w1527 -> [w1535 w1538]
          tunnel: [w1535 w1537] -> w1519
          frame False {
          }
          frame True {
            n945 = Build Array (concatenate)(w1541, w1540) -> (w1539:dbl[][])
            n946 = Build Array (concatenate)(w1538, w1542) -> (w1537:string[])
          }
        }
        "All Labels (USB6210)" <- w1519
        "DataArrayConv (USB6210)" <- w1516
        n947 = control-ref of="Plot selecter (USB6210)\n    1      2     3     4"() -> (w1518:refnum<vi>)
        n948 = local read "Plot selecter (USB6210)\n    1      2     3     4"() -> (w1521:bool[][])
        n949 = Array Size(array=w1519) -> (size(s)=w1532:i32)
        n950 = Array Size(array=w1519) -> (size(s)=w1520:i32)
        n951 = Array Size(array=w1516) -> (size(s)=→"Data Array sizes (6210)":i32[])
        n952 = property on="Property Node" class="Arr (strict)"(reference=w1518, "Number of Rows"=w1520) -> ()  [unwired: 1 in, 2 out]
        n953 = for {
          N: w1532 -> [_]
          tunnel: w1516 -> [w1563]
          tunnel: w1534 -> [w1564]
          shift-right: [w1559] -> w1524
          shift-left: w1525 -> [w1562]
          shift-right: [w1557] -> w1522
          shift-left: w1525 -> [w1560]
          shift-right: [w1558] -> w1526
          shift-left: w1525 -> [w1556]
          shift-right: [w1555] -> w1523
          shift-left: w1525 -> [w1554]
          tunnel: w1521 -> [w1553]
          i -> [w1548]
          n954 = Index Array(array=w1563, index (col)=w1548) -> (element=w1543:dbl[])  [unwired: 1 in]
          n955 = Index Array(array=w1553, index (row) #1=w1548, index (col) #1=0 ("index (row)"), index (row) #2=w1548, index (col) #2=1 ("index (row)"), index (row) #3=w1548, index (col) #3=2 ("index (row)"), index (row) #4=w1548, index (col) #4=3 ("index (row)")) -> (element #1=w1547:bool, element #2=w1546:bool, element #3=w1545:bool, element #4=w1544:bool)
          n956 = Bundle("TimeArray"=w1564, "DataArrayConv"=w1543) -> (w1561:T31)  [unwired: 1 in]
          n957 = stacked-sequence {
            tunnel: w1547 -> [w1568 _ _ _]
            tunnel: w1562 -> [_ w1576 _ _]
            tunnel: w1545 -> [_ _ w1584 _]
            tunnel: w1561 -> [w1565 w1574 w1583 w1589]
            tunnel: w1544 -> [_ _ _ w1592]
            tunnel: w1560 -> [_ _ _ w1591]
            tunnel: [_ _ _ w1590] -> w1557
            tunnel: [_ w1575 _ _] -> w1559
            tunnel: [w1567 _ _ _] -> w1558
            tunnel: w1556 -> [w1566 _ _ _]
            tunnel: [_ _ w1582 _] -> w1555
            tunnel: w1554 -> [_ _ w1581 _]
            tunnel: w1546 -> [_ w1573 _ _]
            frame #0 {
              n958 = case shown="True" w1568 {
                tunnel: [w1569 w1572] -> w1567
                tunnel: w1565 -> [_ w1571]
                tunnel: w1566 -> [w1569 w1570]
                frame False {
                }
                frame True {
                  n959 = Build Array (concatenate)(w1570, w1571) -> (w1572:T25)
                }
              }
            }
            frame #1 {
              n960 = case shown="True" w1573 {
                tunnel: w1576 -> [w1577 w1580]
                tunnel: [w1577 w1579] -> w1575
                tunnel: w1574 -> [_ w1578]
                frame False {
                }
                frame True {
                  n961 = Build Array (concatenate)(w1580, w1578) -> (w1579:T25)
                }
              }
            }
            frame #2 {
              n962 = case shown="True" w1584 {
                tunnel: [w1585 w1588] -> w1582
                tunnel: w1583 -> [_ w1587]
                tunnel: w1581 -> [w1585 w1586]
                frame False {
                }
                frame True {
                  n963 = Build Array (concatenate)(w1586, w1587) -> (w1588:T25)
                }
              }
            }
            frame #3 {
              n964 = case shown="True" w1592 {
                tunnel: [w1593 w1596] -> w1590
                tunnel: w1589 -> [_ w1595]
                tunnel: w1591 -> [w1593 w1594]
                frame False {
                }
                frame True {
                  n965 = Build Array (concatenate)(w1594, w1595) -> (w1596:T25)
                }
              }
            }
          }
        }
      }
    }
    n966 = local read "Plot selecter LSI218(2)\n    1      2     3     4"() -> (w919:bool[][])
    n967 = local read "Plot selecter LSI218(1)\n    1      2     3     4"() -> (w920:bool[][])
    n968 = for {
      N: 48 -> [_]
      tunnel: w935 -> [w1985]
      tunnel: w934 -> [w1982]
      tunnel: w920 -> [w1966]
      tunnel: w919 -> [w1967]
      shift-right: [w1983] -> w933
      shift-left: w931 -> [w1984]
      shift-right: [w1978] -> w928
      shift-left: w931 -> [w1979]
      shift-right: [w1977] -> w926
      shift-left: w931 -> [w1976]
      shift-right: [w1975] -> w924
      shift-left: w931 -> [w1974]
      i -> [w1972]
      n969 = Index Array(array=w1982, index (col)=w1972) -> (element=w1981:dbl[])  [unwired: 1 in]
      n970 = Less?(x=w1972, y=24) -> (x < y?=w1973:bool)
      n971 = case shown="True" w1973 {
        tunnel: [w1990 w2008] -> w1971
        tunnel: [w1989 w2007] -> w1970
        tunnel: [w1988 w2005] -> w1969
        tunnel: [w1987 w2004] -> w1968
        tunnel: w1966 -> [_ w2003]
        tunnel: w1967 -> [w1997 _]
        tunnel: w1972 -> [w1992 w2000]
        frame False {
          n972 = Subtract(x=w1992, y=24) -> (x-y=w1996:i32)
          n973 = Index Array(array=w1997, index (row) #1=w1996, index (col) #1=0 ("index (row)"), index (row) #2=w1996, index (col) #2=1 ("index (row)"), index (row) #3=w1996, index (col) #3=2 ("index (row)"), index (row) #4=w1996, index (col) #4=3 ("index (row)")) -> (element #1=w1990:bool, element #2=w1989:bool, element #3=w1988:bool, element #4=w1987:bool)
        }
        frame True {
          n974 = Index Array(array=w2003, index (row) #1=w2000, index (col) #1=0 ("index (row)"), index (row) #2=w2000, index (col) #2=1 ("index (row)"), index (row) #3=w2000, index (col) #3=2 ("index (row)"), index (row) #4=w2000, index (col) #4=3 ("index (row)")) -> (element #1=w2008:bool, element #2=w2007:bool, element #3=w2005:bool, element #4=w2004:bool)
        }
      }
      n975 = Bundle("TimeArray"=w1985, "DataArray"=w1981) -> (w1980:T35)  [unwired: 1 in]
      n976 = stacked-sequence {
        tunnel: w1984 -> [w2012 _ _ _]
        tunnel: [w2011 _ _ _] -> w1983
        tunnel: w1980 -> [w2010 w2020 w2028 w2036]
        tunnel: w1979 -> [_ w2019 _ _]
        tunnel: [_ w2018 _ _] -> w1978
        tunnel: [_ _ w2027 _] -> w1977
        tunnel: w1976 -> [_ _ w2026 _]
        tunnel: [_ _ _ w2035] -> w1975
        tunnel: w1974 -> [_ _ _ w2034]
        tunnel: w1971 -> [w2009 _ _ _]
        tunnel: w1970 -> [_ w2017 _ _]
        tunnel: w1969 -> [_ _ w2025 _]
        tunnel: w1968 -> [_ _ _ w2033]
        frame #0 {
          n977 = case shown="False" w2009 {
            tunnel: w2010 -> [_ w2014]
            tunnel: w2012 -> [w2013 w2016]
            tunnel: [w2013 w2015] -> w2011
            frame False {
            }
            frame True {
              n978 = Build Array (concatenate)(w2016, w2014) -> (w2015:T4)
            }
          }
        }
        frame #1 {
          n979 = case shown="True" w2017 {
            tunnel: [w2021 w2024] -> w2018
            tunnel: w2020 -> [_ w2023]
            tunnel: w2019 -> [w2021 w2022]
            frame False {
            }
            frame True {
              n980 = Build Array (concatenate)(w2022, w2023) -> (w2024:T4)
            }
          }
        }
        frame #2 {
          n981 = case shown="True" w2025 {
            tunnel: [w2029 w2032] -> w2027
            tunnel: w2028 -> [_ w2031]
            tunnel: w2026 -> [w2029 w2030]
            frame False {
            }
            frame True {
              n982 = Build Array (concatenate)(w2030, w2031) -> (w2032:T4)
            }
          }
        }
        frame #3 {
          n983 = case shown="True" w2033 {
            tunnel: [w2037 w2040] -> w2035
            tunnel: w2036 -> [_ w2039]
            tunnel: w2034 -> [w2037 w2038]
            frame False {
            }
            frame True {
              n984 = Build Array (concatenate)(w2038, w2039) -> (w2040:T4)
            }
          }
        }
      }
    }
    n985 = local read "Labels LSI336"() -> (w907:string[])
    n986 = Array Size(array=w907) -> (size(s)=w906:i32)
    n987 = local read "Plot selecter LSI336 \n     1      2     3     4"() -> (w915:bool[][])
    n988 = for {
      N: w906 -> [_]
      tunnel: w915 -> [w1898]
      shift-right: [w1892] -> w913
      shift-left: w914 -> [w1907]
      shift-right: [w1888] -> w912
      shift-left: w914 -> [w1905]
      shift-right: [w1889] -> w911
      shift-left: w914 -> [w1904]
      shift-right: [w1887] -> w910
      shift-left: w914 -> [w1903]
      tunnel: w876 -> [w1895]
      tunnel: w878 -> [w1893]
      i -> [w1896]
      n989 = Index Array(array=w1895, index (col)=w1896) -> (element=w1894:dbl[])  [unwired: 1 in]
      n990 = Index Array(array=w1898, index (row) #1=w1896, index (col) #1=0 ("index (row)"), index (row) #2=w1896, index (col) #2=1 ("index (row)"), index (row) #3=w1896, index (col) #3=2 ("index (row)"), index (row) #4=w1896, index (col) #4=3 ("index (row)")) -> (element #1=w1897:bool, element #2=w1891:bool, element #3=w1890:bool, element #4=w1886:bool)
      n991 = Bundle("TimeArray"=w1893, "DataArray"=w1894) -> (w1906:T35)  [unwired: 1 in]
      n992 = stacked-sequence {
        tunnel: w1907 -> [w1911 _ _ _]
        tunnel: [w1910 _ _ _] -> w1892
        tunnel: w1906 -> [w1909 w1919 w1927 w1935]
        tunnel: w1905 -> [_ w1918 _ _]
        tunnel: [_ w1917 _ _] -> w1888
        tunnel: [_ _ w1926 _] -> w1889
        tunnel: w1904 -> [_ _ w1925 _]
        tunnel: [_ _ _ w1934] -> w1887
        tunnel: w1903 -> [_ _ _ w1933]
        tunnel: w1897 -> [w1908 _ _ _]
        tunnel: w1891 -> [_ w1916 _ _]
        tunnel: w1890 -> [_ _ w1924 _]
        tunnel: w1886 -> [_ _ _ w1932]
        frame #0 {
          n993 = case shown="False" w1908 {
            tunnel: w1909 -> [_ w1913]
            tunnel: w1911 -> [w1912 w1915]
            tunnel: [w1912 w1914] -> w1910
            frame False {
            }
            frame True {
              n994 = Build Array (concatenate)(w1915, w1913) -> (w1914:T4)
            }
          }
        }
        frame #1 {
          n995 = case shown="True" w1916 {
            tunnel: [w1920 w1923] -> w1917
            tunnel: w1919 -> [_ w1921]
            tunnel: w1918 -> [w1920 w1922]
            frame False {
            }
            frame True {
              n996 = Build Array (concatenate)(w1922, w1921) -> (w1923:T4)
            }
          }
        }
        frame #2 {
          n997 = case shown="True" w1924 {
            tunnel: [w1928 w1931] -> w1926
            tunnel: w1927 -> [_ w1929]
            tunnel: w1925 -> [w1928 w1930]
            frame False {
            }
            frame True {
              n998 = Build Array (concatenate)(w1930, w1929) -> (w1931:T4)
            }
          }
        }
        frame #3 {
          n999 = case shown="True" w1932 {
            tunnel: [w1936 w1939] -> w1934
            tunnel: w1935 -> [_ w1937]
            tunnel: w1933 -> [w1936 w1938]
            frame False {
            }
            frame True {
              n1000 = Build Array (concatenate)(w1938, w1937) -> (w1939:T4)
            }
          }
        }
      }
    }
    n1001 = Array Size(array=w878) -> (size(s)=→"TimeArray Size (336)":i32)
    n1002 = Array Size(array=w876) -> (size(s)=→"DataArray size (336)":i32[])
    n1003 = Build Array (concatenate)(w932, w933, w913, w891, w836) -> (→"Graph 1":T25)
    n1004 = Build Array (concatenate)(w930, w928, w912, w890, w835) -> (→"Graph 2":T25)
    n1005 = Build Array (concatenate)(w927, w926, w911, w889, w834) -> (→"Graph 3":T25)
    n1006 = Build Array (concatenate)(w925, w924, w910, w888, w833) -> (→"Graph 4":T25)
    n1007 = Send Notification(notification="Stop Button", notifier=w853, error in (no error)=w852) -> (notifier out=w849:refnum<notifier>, error out=w850:errorcluster)